vi "字符图片截取.vi"(8 "error in (no error)":errorcluster, 10 "Optional Rectangle":i32[](array[numeric])=[1531, 590, 2568, 1924], 11 "Image":T1(plugin-control)=refnum) -> (0 "error out":errorcluster, 2 "Image 2":T1(plugin-control), 3 "Image 3":T1(plugin-control))   [LabVIEW 2017]
uses:
  <vilib>/vision/NI_Vision_Development_Module.lvlib
panel:
  in  "Optional Rectangle 2":i32[](array[numeric])=[1658, 727, 2568, 1924]
  out "X Resolution":i32=1037
  out "Y Resolution":i32=1334
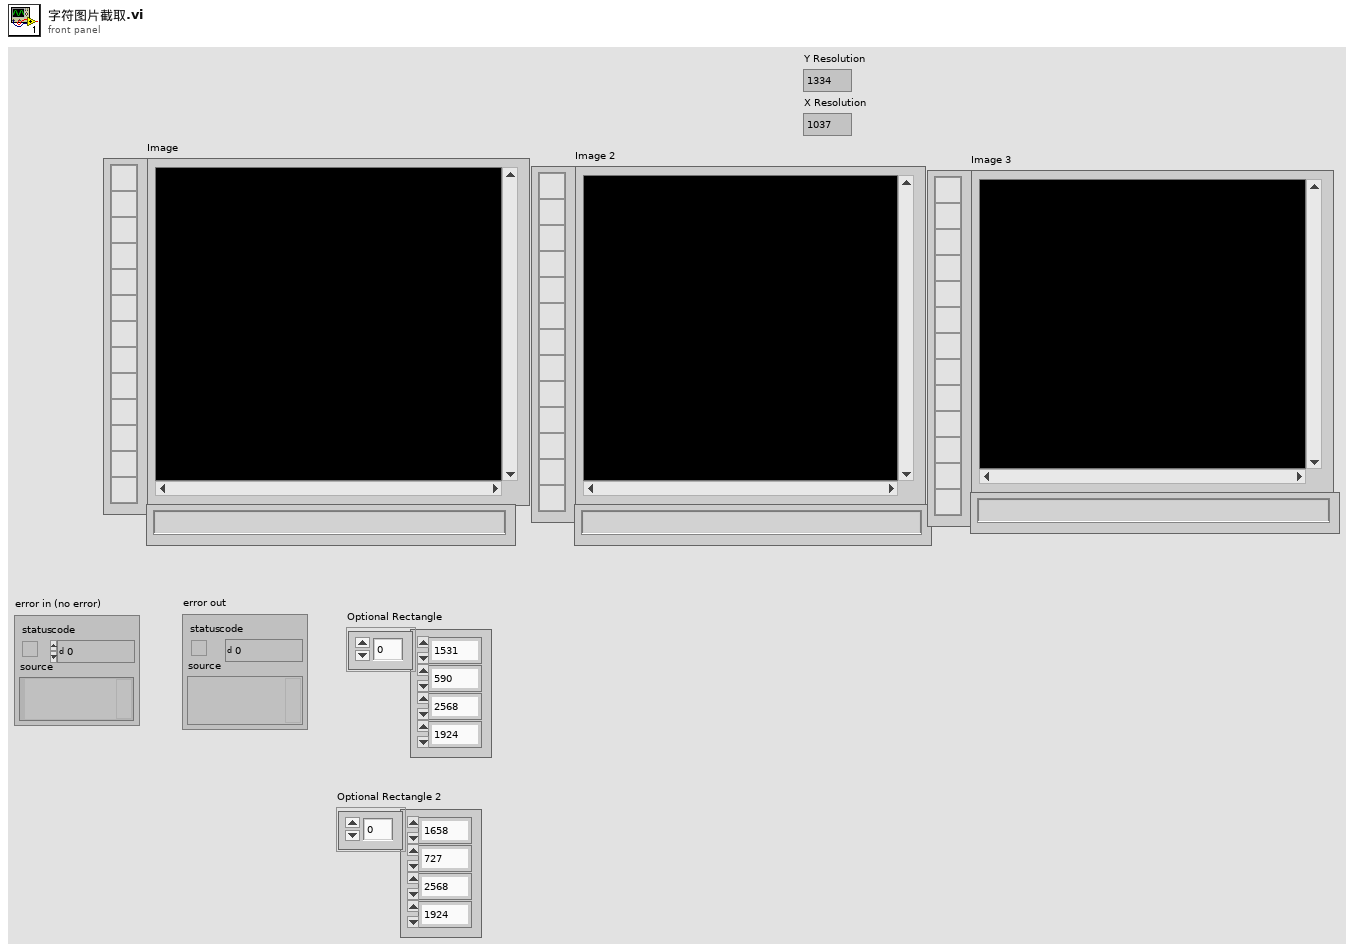
[diagram p1: front panel]
types:
  T1 = typedef "IMAQ Image.ctl" = refnum<image>
  T2 = typedef "Image Type" = u32
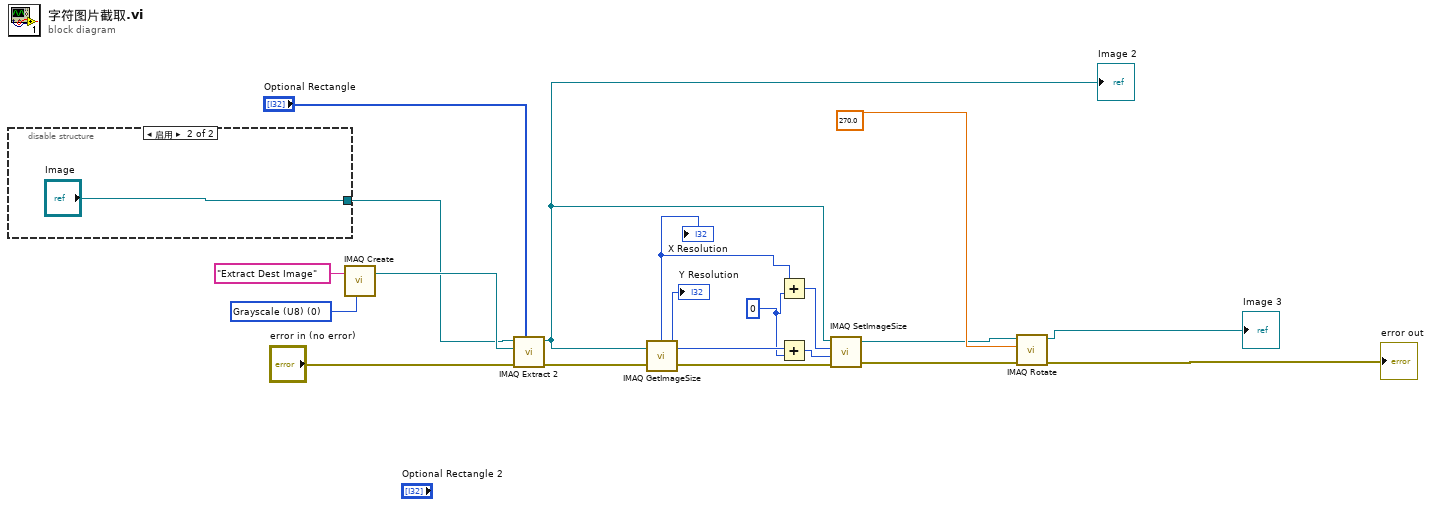
[diagram p0: block diagram]
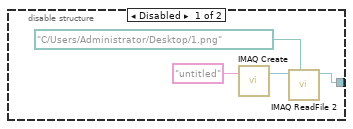
[diagram p2: hidden frame]
diagram:
  w1 = 0 ("y")
  w18 = T2 0 items=["Grayscale (U8)", "Grayscale (I16)", "Grayscale (SGL)", "Complex (CSG)", "RGB (U32)", "HSL (U32)", "RGB (U64)", "Grayscale (U16)"] ("Image Type")
  n1 = disable-structure shown="启用" {
    disable-tunnel: [w20 "Image"] -> w9
    frame Disabled {
      n2 = call "IMAQ Create"("Image Name"="untitled") -> ("New Image"=w22:T1)  [unwired: 4 in, 1 out]
      n3 = call "IMAQ ReadFile 2"("File Path"=path "C:/Users/Administrator/Desktop/1.png", "Image"=w22) -> ("Image Out"=w20:T1)  [unwired: 5 in, 4 out]
    }
    frame Enabled {
    }
  }
  n4 = call "IMAQ Create"("Image Name"="Extract Dest Image", "Image Type"=w18) -> ("New Image"=w15:T1)  [unwired: 3 in, 1 out]
  n5 = call "IMAQ Extract 2"("Optional Rectangle"="Optional Rectangle", "error in (no error)"="error in (no error)", "Image Dst"=w15, "Image Src"=w9) -> ("error out"=w12:errorcluster, "Image Dst Out"=w10:T1)  [unwired: 6 in]
  "Image 2" <- w10
  n6 = call "IMAQ GetImageSize"("Image"=w10, "error in (no error)"=w12) -> ("Y Resolution"=w5:i32, "X Resolution"=w6:i32, "error out"=w7:errorcluster)  [unwired: 2 in]
  "Y Resolution" <- w5
  "X Resolution" <- w6
  n7 = Add(x=w6, y=w1) -> (x+y=w4:i32)
  n8 = Add(x=w5, y=w1) -> (x+y=w3:i32)
  n9 = call "IMAQ SetImageSize"("error in (no error)"=w7, "Y Resolution"=w3, "X Resolution"=w4, "Image"=w10) -> ("error out"=w13:errorcluster, "Image Out"=w2:T1)  [unwired: 1 in]
  n10 = call "IMAQ Rotate"("error in (no error)"=w13, "Angle (degrees)"=sgl 270.0, "Image Src"=w2) -> ("error out"=→"error out":errorcluster, "Image Dst Out"=→"Image 3":T1)  [unwired: 7 in]
